vi "Diseño_SCADA_Con_gases.vi"() -> ()   [LabVIEW 2024]
panel:
  in  "stop":bool
  in  "Tab Control":T1(tab)
  out "E2.1.2":bool caption="Not initialized"
  out "E1.1":bool caption="Maintenance mode"
  out "E2.2.2":bool caption="Not initialized"
  out "E2.3.2":bool caption="Not initialized"
  out "E1.2.2":bool caption="Maintenance mode"
  out "E1.3.2":bool caption="Idle"
  out "Humedad":dbl format="%#.4g"
  out "Temperatura":dbl format="%#.4g"
  out "Prod electrolizadores (display) 2":dbl format="%#.4g"
  out "Potenica Solar (Display) 2":dbl format="%#.2f"
  out "masa total G Kg 2":dbl format="%#.3f"
  out "P alta 2":dbl format="%.1f"
  out "P baja 2":dbl format="%.1f"
  out "masa total P Kg  2":dbl format="%#.3f"
  in  "SAI":bool caption="Line"
  out "Potenica SAI (Display) 3":dbl format="%#.2f"
  out "Comunicacion SAI":bool
  out "E2.1":bool caption="Not initialized"
  out "E2.2":bool caption="Not initialized"
  out "E1.3":bool caption="Idle"
  out "E1.1,2":bool caption="Maintenance mode"
  out "E2.3":bool caption="Not initialized"
  out "E1.2":bool caption="Maintenance mode"
  out "Producció d'hidrogen":dbl(graph)
  out "Energia solar no utilitzada":dbl(graph)
  out "Pressió tanc baixa":dynamicdata(graph)
  out "Potenica Solar (Display)":dbl format="%#.2f"
  out "Producción FC":dbl format="%#_2g"
  out "Prod electrolizadores (display)":dbl format="%#.4g"
  out "P baja":dbl format="%.1f"
  out "masa total G Kg":dbl format="%#.0f"
  out "Potència inversor solar":dynamicdata(graph)
  out "Watimetro ARPA":dbl format="%#.1f"
  out "masa total P Kg":dbl format="%#.1f"
  out "Compresor":bool
  out "P alta":dbl format="%.1f"
  out "Tèrmic\nExtractors":bool
  out "Relé Seguretat":bool
  out "Sobretensions":bool
  out "Baliza verde":bool
  out "Baliza amarilla":bool
  out "Baliza roja":bool
  out "H2 generado Total":dbl format="%#.1f"
  out "Producción Solar toral":dbl format="%#.1f"
  out "Energía acum H2 verde":dbl format="%#.1f"
  out "H2 consumido en el lab":dbl=182.6 format="%#.1f"
  out "Energía solar diaría":dbl format="%#.1f"
  out "H2 generado dia":dbl format="%#.1f"
  out "Comunicacion Inversor SALICRU":bool
  out "Tank":dbl(slide) scale=0.0..10.0
  out "CO":dbl format="%.1f"
  out "NO2":dbl format="%#.3f"
  out "O3":dbl format="%.1f"
  out "SO2":dbl format="%#.3f"
  out "CO2":dbl format="%.1f"
  out "O2":dbl format="%#.3f"
  out "TVOC":dbl format="%.1f"
  out "H2S":dbl format="%#.3f"
  out "Qualitat de l'aire":dbl[](graph)
  # "Ambiente"
  # "Temperatura"
  # "ºC"
  # "Humedad"
  # "%"
  # "ESTADO ELY"
  # "E1.1"
  # "E2.1"
  # "E1.2"
  # "E2.2"
  # "E2.3"
  # "E1.3"
  # "Modo:"
  # "RESUMEN DE LA PRODUCCIÓN"
  # "SAI PLANTA"
  # "Electrolizadores"
  # "Producción\nElectrolizadores:"
  # "g/s"
  # "Inversor solar:"
  # "Energía solar:"
  # "kW"
  # "Tanque Alta"
  # "Presión:"
  # "barg"
  # "Kg"
  # "Capacidad:"
  # "Tanque Baja"
  # "Presión:"
  # "barg"
  # "Kg"
  # "Capacidad:"
  # "SAI:"
  # "Potencia (%):"
  # "%"
  # "Seguretat"
  # "Hidrògen"
  # "H2 baixa pressió"
  # "H2 alta pressió"
  # "Aigua"
  # "barg"
  # "Tanc baixa pressió"
  # "Tanc alta pressió"
  # "Compressor"
  # "barg"
  # "Solar"
  # "Fuel Cell"
  # "kW"
  # "kW"
  # "kg"
  # "kg"
  # "Electrolizadors"
  # "g/s"
  # "Xarxa electrica"
  # "-"
  # "+"
  # "kW de xarxa"
  # "Producció total d'hidrogen"
  # "Producció d'hidrogen diària"
  # "g"
  # "kg"
  # "Producció total d'energia solar"
  # "Energia solar produïda diària"
  # "kWh"
  # "kWh"
  # "Energia acumulada per H2 verd"
  # "Consum de H2 Lab diari"
  # "g"
  # "kWh"
  # "Gases"
  # "ppm"
  # "TVOC:"
  # "ppm"
  # "H2S:"
  # "ppm"
  # "CO2:"
  # "ppm"
  # "O2:"
  # "ppm"
  # "O3:"
  # "ppm"
  # "SO2:"
  # "ppm"
  # "CO:"
  # "ppm"
  # "NO2:"
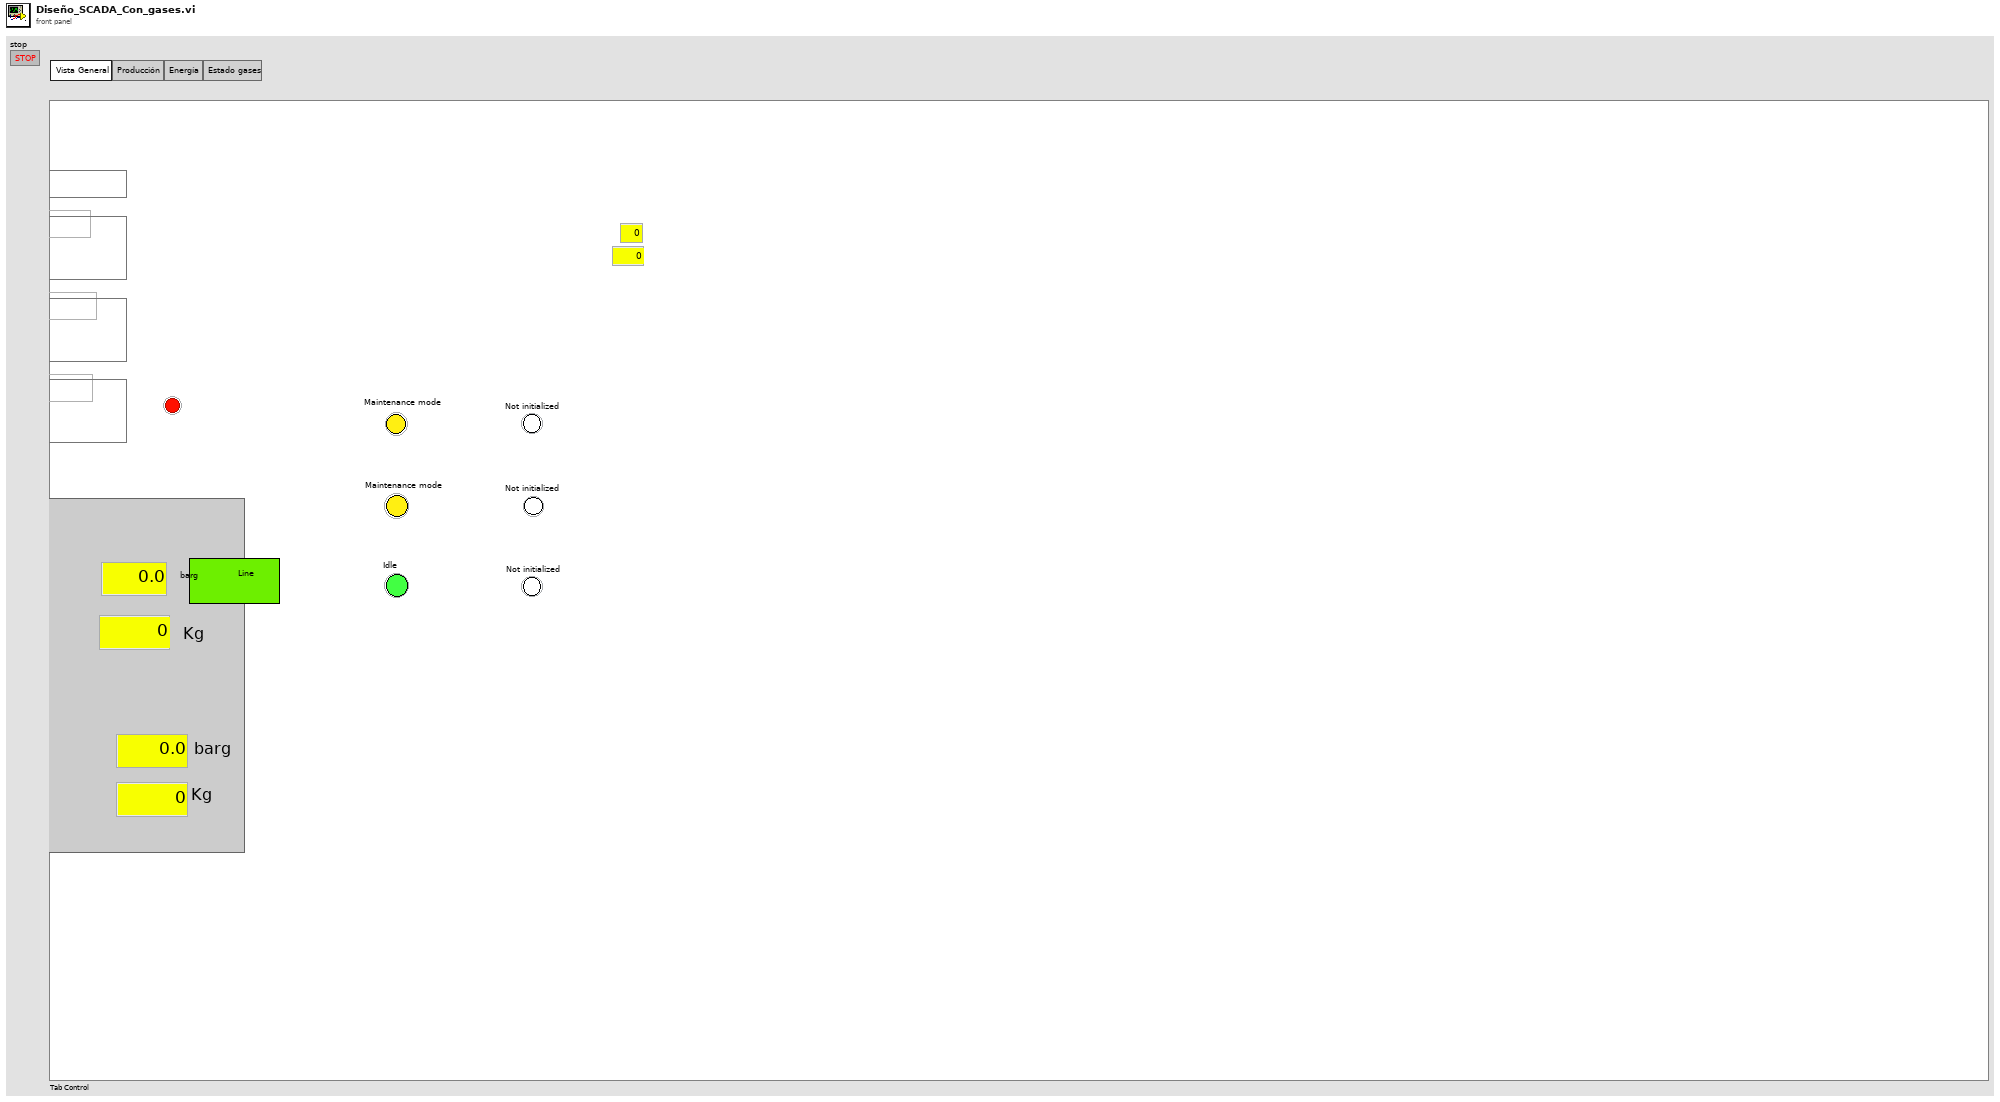
[diagram p1: front panel]
types:
  T1 = enum32{"Vista General", "Producción", "Energía", "Estado gases"}
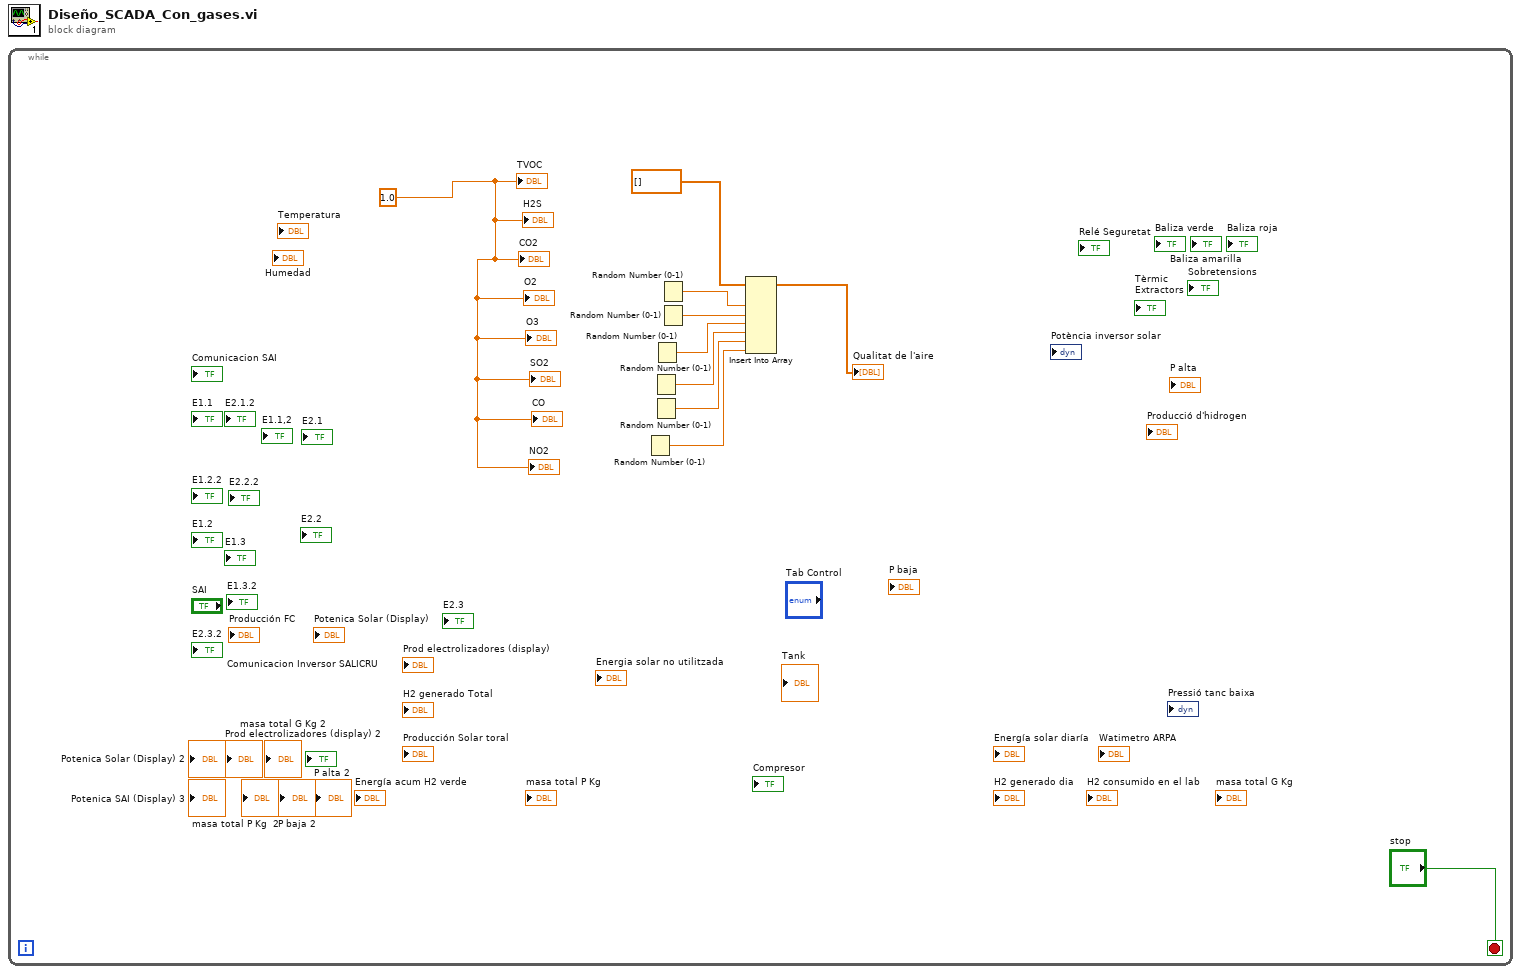
[diagram p0: block diagram]
diagram:
  n1 = while {
    stop <- "stop" stop-if-true
    w9 = 1.0 ("TVOC")
    n2 = Random Number (0-1)() -> (number: 0 to 1=w1:dbl)
    n3 = Random Number (0-1)() -> (number: 0 to 1=w3:dbl)
    n4 = Random Number (0-1)() -> (number: 0 to 1=w2:dbl)
    n5 = Random Number (0-1)() -> (number: 0 to 1=w4:dbl)
    n6 = Random Number (0-1)() -> (number: 0 to 1=w6:dbl)
    n7 = Random Number (0-1)() -> (number: 0 to 1=w5:dbl)
    n8 = Insert Into Array(array=dbl[] [], new element #1=w6, new element #2=w5, new element #3=w4, new element #4=w3, new element #5=w2, new element #6=w1) -> (→"Qualitat de l'aire":dbl[])  [unwired: 1 in]
    "H2S" <- w9
    "TVOC" <- w9
    "O2" <- w9
    "CO2" <- w9
    "SO2" <- w9
    "O3" <- w9
    "NO2" <- w9
    "CO" <- w9
  }
